vi "CRYO_MASTER_FULL_RUN3.vi"() -> ()   [LabVIEW 2017] (continued)
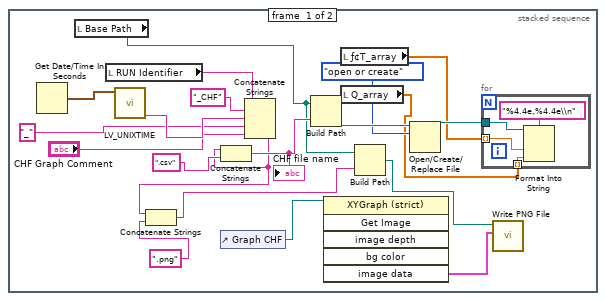
[diagram p3: hidden frame]
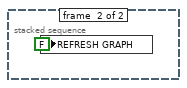
[diagram p5: hidden frame]
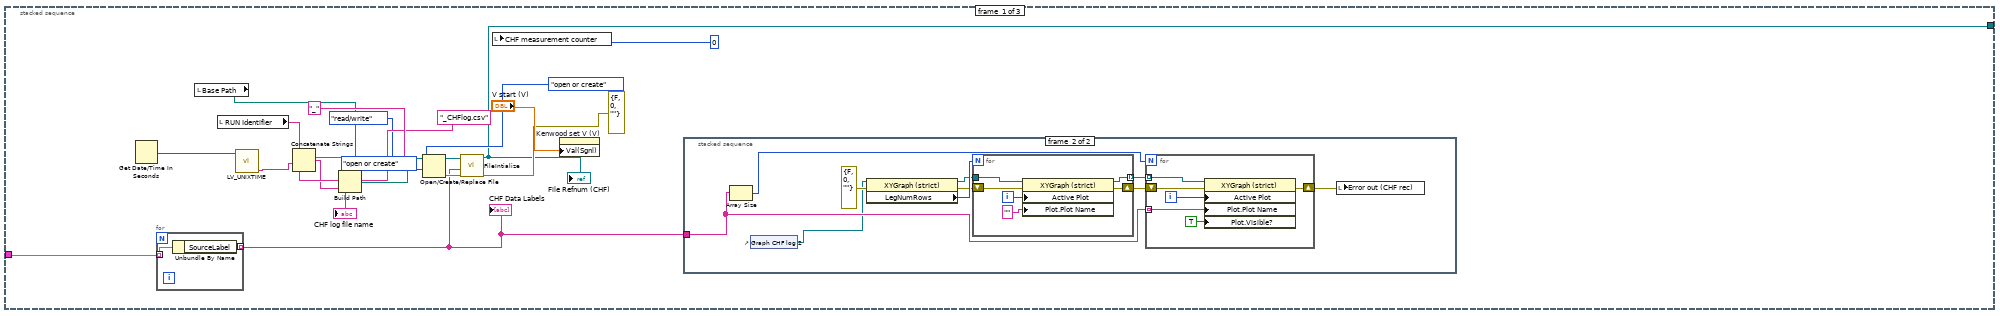
[diagram p7: hidden frame]
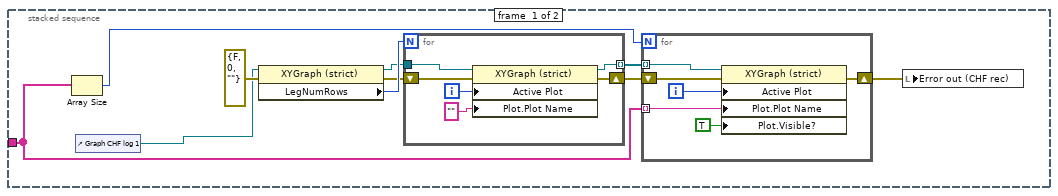
[diagram p8: hidden frame]
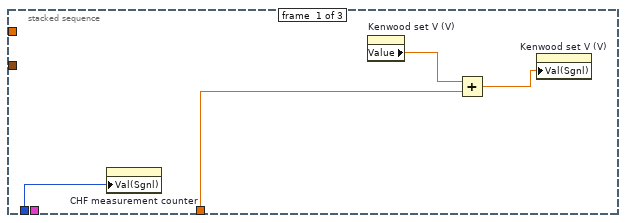
[diagram p9: hidden frame]
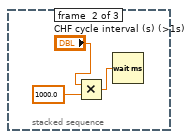
[diagram p10: hidden frame]
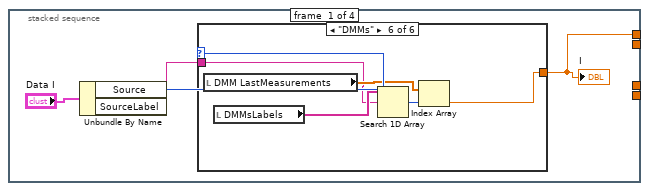
[diagram p11: hidden frame]
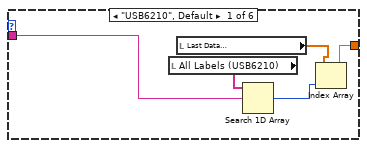
[diagram p12: hidden frame]
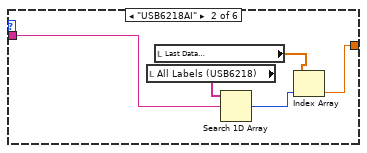
[diagram p13: hidden frame]
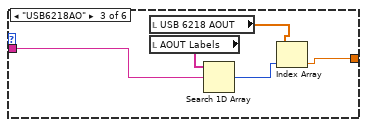
[diagram p14: hidden frame]
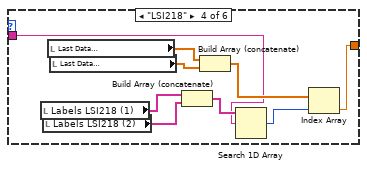
[diagram p15: hidden frame]
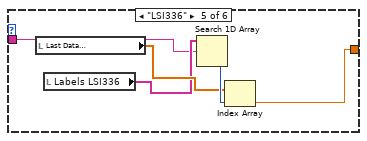
[diagram p16: hidden frame]
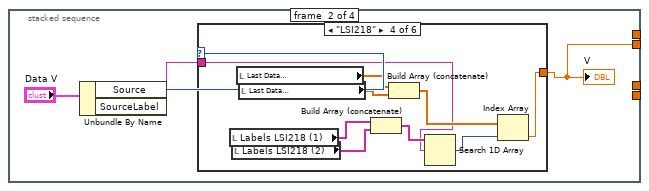
[diagram p17: hidden frame]
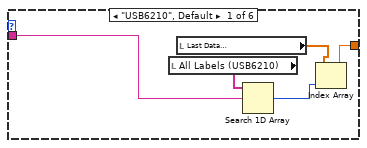
[diagram p18: hidden frame]
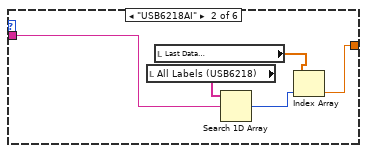
[diagram p19: hidden frame]
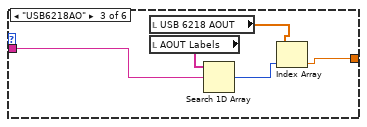
[diagram p20: hidden frame]
            frame False {
            }
            frame True {
              n984 = Build Array (concatenate)(w2040, w2041) -> (w2042:T4)
            }
          }
        }
      }
    }
    n985 = local read "Labels LSI336"() -> (w907:string[])
    n986 = Array Size(array=w907) -> (size(s)=w906:i32)
    n987 = local read "Plot selecter LSI336 \n     1      2     3     4"() -> (w915:bool[][])
    n988 = for {
      N: w906 -> [_]
      tunnel: w915 -> [w1900]
      shift-right: [w1894] -> w913
      shift-left: w914 -> [w1909]
      shift-right: [w1890] -> w912
      shift-left: w914 -> [w1907]
      shift-right: [w1891] -> w911
      shift-left: w914 -> [w1906]
      shift-right: [w1889] -> w910
      shift-left: w914 -> [w1905]
      tunnel: w876 -> [w1897]
      tunnel: w878 -> [w1895]
      i -> [w1898]
      n989 = Index Array(array=w1897, index (col)=w1898) -> (element=w1896:dbl[])  [unwired: 1 in]
      n990 = Index Array(array=w1900, index (row) #1=w1898, index (col) #1=0 ("index (row)"), index (row) #2=w1898, index (col) #2=1 ("index (row)"), index (row) #3=w1898, index (col) #3=2 ("index (row)"), index (row) #4=w1898, index (col) #4=3 ("index (row)")) -> (element #1=w1899:bool, element #2=w1893:bool, element #3=w1892:bool, element #4=w1888:bool)
      n991 = Bundle("TimeArray"=w1895, "DataArray"=w1896) -> (w1908:T35)  [unwired: 1 in]
      n992 = stacked-sequence {
        tunnel: w1909 -> [w1913 _ _ _]
        tunnel: [w1912 _ _ _] -> w1894
        tunnel: w1908 -> [w1911 w1921 w1929 w1937]
        tunnel: w1907 -> [_ w1920 _ _]
        tunnel: [_ w1919 _ _] -> w1890
        tunnel: [_ _ w1928 _] -> w1891
        tunnel: w1906 -> [_ _ w1927 _]
        tunnel: [_ _ _ w1936] -> w1889
        tunnel: w1905 -> [_ _ _ w1935]
        tunnel: w1899 -> [w1910 _ _ _]
        tunnel: w1893 -> [_ w1918 _ _]
        tunnel: w1892 -> [_ _ w1926 _]
        tunnel: w1888 -> [_ _ _ w1934]
        frame #0 {
          n993 = case shown="False" w1910 {
            tunnel: w1911 -> [_ w1915]
            tunnel: w1913 -> [w1914 w1917]
            tunnel: [w1914 w1916] -> w1912
            frame False {
            }
            frame True {
              n994 = Build Array (concatenate)(w1917, w1915) -> (w1916:T4)
            }
          }
        }
        frame #1 {
          n995 = case shown="True" w1918 {
            tunnel: [w1922 w1925] -> w1919
            tunnel: w1921 -> [_ w1923]
            tunnel: w1920 -> [w1922 w1924]
            frame False {
            }
            frame True {
              n996 = Build Array (concatenate)(w1924, w1923) -> (w1925:T4)
            }
          }
        }
        frame #2 {
          n997 = case shown="True" w1926 {
            tunnel: [w1930 w1933] -> w1928
            tunnel: w1929 -> [_ w1931]
            tunnel: w1927 -> [w1930 w1932]
            frame False {
            }
            frame True {
              n998 = Build Array (concatenate)(w1932, w1931) -> (w1933:T4)
            }
          }
        }
        frame #3 {
          n999 = case shown="True" w1934 {
            tunnel: [w1938 w1941] -> w1936
            tunnel: w1937 -> [_ w1939]
            tunnel: w1935 -> [w1938 w1940]
            frame False {
            }
            frame True {
              n1000 = Build Array (concatenate)(w1940, w1939) -> (w1941:T4)
            }
          }
        }
      }
    }
    n1001 = Array Size(array=w878) -> (size(s)=→"TimeArray Size (336)":i32)
    n1002 = Array Size(array=w876) -> (size(s)=→"DataArray size (336)":i32[])
    n1003 = Build Array (concatenate)(w932, w933, w913, w891, w836) -> (→"Graph 1":T25)
    n1004 = Build Array (concatenate)(w930, w928, w912, w890, w835) -> (→"Graph 2":T25)
    n1005 = Build Array (concatenate)(w927, w926, w911, w889, w834) -> (→"Graph 3":T25)
    n1006 = Build Array (concatenate)(w925, w924, w910, w888, w833) -> (→"Graph 4":T25)
    n1007 = Send Notification(notification="Stop Button", notifier=w853, error in (no error)=w852) -> (notifier out=w849:refnum<notifier>, error out=w850:errorcluster)
    "Cycle #" <- w842
  }
  n1008 = while {
    tunnel: w5 -> [w2130]
    tunnel: w4 -> [w2129]
    stop <- w2131 stop-if-true
    n1009 = Wait (ms)(milliseconds to wait=u32 214) -> ()  [unwired: 1 out]
    n1010 = case shown="True" "RECORD GRAPH" {
      frame False {
      }
      frame True {
        n1011 = stacked-sequence {
          frame #0 {
            n1012 = Get Date/Time In Seconds() -> (seconds since 1Jan1904=w2152:timestamp)
            n1013 = local read "Base Path"() -> (w2137:path)
            n1014 = local read "RUN Identifier"() -> (w2153:string)
            n1015 = call "LV_UNIXTIME.vi"("current time"=w2152) -> ("date/time string"=w2154:string)  [unwired: 9 in, 1 out]
            n1016 = control-ref of="Graph CHF"() -> (w2143:refnum<vi>)
            n1017 = Concatenate Strings(w2153, "_CHF" ("string"), w2154, "_" ("string"), "CHF Graph Comment") -> (w2139:string)
            n1018 = Concatenate Strings(w2139, ".png" ("string")) -> (w2138:string)
            n1019 = Concatenate Strings(w2139, ".csv" ("string")) -> (w2141:string)
            "CHF file name" <- w2141
            n1020 = Build Path(base path=w2137, name or relative path=w2141) -> (appended path=w2148:path)
            n1021 = invoke class="XYGraph (strict)" method="Get Image"(reference=w2143) -> ("image data"=w2135:T23)  [unwired: 5 in, 5 out]
            n1022 = local read "ƒ¢T_array"() -> (w2145:dbl[])
            n1023 = local read "Q_array"() -> (w2144:dbl[])
            n1024 = Build Path(base path=w2137, name or relative path=w2138) -> (appended path=w2136:path)
            n1025 = Open/Create/Replace File(file path (use dialog)=w2148, operation (0:open)=T24."open or create") -> (refnum out=w2146:refnum<file>)  [unwired: 4 in, 2 out]
            n1026 = for {
              tunnel: w2146 -> [w2158]
              tunnel: w2145 -> [w2156] mode=indexing
              tunnel: w2144 -> [w2155] mode=indexing
              n1027 = Format Into String(format string="%4.4e,%4.4e\\n" ("prompt"), initial string=w2158, w2156, w2155) -> ()  [unwired: 1 in, 2 out]
            }
            n1028 = call <vilib>:"Write PNG File.vi"("image data"=w2135, "path to PNG file"=w2136) -> ()  [unwired: 8 in, 2 out]
          }
          frame #1 {
            n1029 = local write "RECORD GRAPH"(FALSE ("RECORD GRAPH")) -> ()
          }
        }
      }
    }
    n1030 = case shown="True" "START CHF" {
      tunnel: "RecordSettings" -> [_ w2163]
      frame False {
      }
      frame True {
        n1031 = stacked-sequence {
          tunnel: [w2167 _ _] -> _
          tunnel: w2163 -> [w2166 w2240 _]
          frame #0 {
            (unwired) T24."open or create" ("operation (0:open)")
            n1032 = Get Date/Time In Seconds() -> (seconds since 1Jan1904=w2179:timestamp)
            n1033 = for {
              tunnel: [w2227] -> w2165 mode=indexing
              tunnel: w2166 -> [w2226] mode=indexing
              n1034 = Unbundle By Name(w2226) -> ("SourceLabel"=w2227:string)
            }
            "CHF Data Labels" <- w2165
            n1035 = local read "Base Path"() -> (w2174:path)
            n1036 = local read "RUN Identifier"() -> (w2178:string)
            n1037 = call "LV_UNIXTIME.vi"("current time"=w2179) -> ("date/time string"=w2177:string)  [unwired: 9 in, 1 out]
            n1038 = Concatenate Strings(w2178, "_" ("string"), w2177, "_CHFlog.csv" ("string")) -> (w2173:string)
            "CHF log file name" <- w2173
            n1039 = Build Path(base path=w2174, name or relative path=w2173) -> (appended path=w2172:path)
            n1040 = Open/Create/Replace File(file path (use dialog)=w2172, error in=errorcluster {"status"=FALSE, "code"=0, "source"=""}, operation (0:open)=T24."open or create", access (0:read/write)=enum16{"read/write", "read-only", "write-only"}."read/write") -> (refnum out=w2170:refnum<file>, error out=w2169:errorcluster)  [unwired: 2 in, 1 out]
            n1041 = call "FileIntialize.vi"("Error In"=w2169, "Labels"=w2165, "refnum in"=w2170) -> ("File Refnum"=w2167:refnum<file>)  [unwired: 7 in, 1 out]
            "File Refnum (CHF)" <- w2167
            n1042 = local write "CHF measurement counter"(0 ("CHF counter")) -> ()
            n1043 = property on="Kenwood set V (V)" class="DigNum (strict)"("Val(Sgnl)"="V start (V)") -> ()  [unwired: 2 in, 2 out]
            n1044 = stacked-sequence {
              tunnel: w2165 -> [w2183 w2206]
              frame #0 {
                n1045 = Array Size(array=w2183) -> (size(s)=w2191:i32)
                n1046 = control-ref of="Graph CHF log 1"() -> (w2184:refnum<vi>)
                n1047 = property class="XYGraph (strict)"(reference=w2184, error in=errorcluster {"status"=FALSE, "code"=0, "source"=""} ("error in (no error)")) -> (reference out=w2186:refnum<vi>, error out=w2188:errorcluster, "LegNumRows"=w2189:u32)
                n1048 = for {
                  N: w2189 -> [_]
                  shift-right: [w2200] -> w2190
                  shift-left: w2188 -> [w2201]
                  tunnel: w2186 -> [w2199]
                  tunnel: [w2198] -> w2185 mode=indexing
                  i -> [w2203]
                  n1049 = property class="XYGraph (strict)"(reference=w2199, error in=w2201, "Active Plot"=w2203, "Plot.Plot Name"="") -> (reference out=w2198:refnum<vi>, error out=w2200:errorcluster)
                }
                n1050 = for {
                  N: w2191 -> [_]
                  shift-right: [w2195] -> w2182
                  shift-left: w2190 -> [w2196]
                  tunnel: w2185 -> [w2193] mode=indexing
                  tunnel: w2183 -> [w2192] mode=indexing
                  i -> [w2197]
                  n1051 = property class="XYGraph (strict)"(reference=w2193, error in=w2196, "Active Plot"=w2197, "Plot.Plot Name"=w2192, "Plot.Visible?"=TRUE ("Plot.Visible")) -> (error out=w2195:errorcluster)  [unwired: 1 out]
                }
                n1052 = local write "Error out (CHF rec)"(w2182) -> ()
              }
              frame #1 {
                n1053 = Array Size(array=w2206) -> (size(s)=w2213:i32)
                n1054 = control-ref of="Graph CHF log 2"() -> (w2205:refnum<vi>)
                n1055 = property class="XYGraph (strict)"(reference=w2205, error in=errorcluster {"status"=FALSE, "code"=0, "source"=""} ("error in (no error)")) -> (reference out=w2208:refnum<vi>, error out=w2210:errorcluster, "LegNumRows"=w2211:u32)
                n1056 = for {
                  N: w2211 -> [_]
                  shift-right: [w2222] -> w2212
                  shift-left: w2210 -> [w2223]
                  tunnel: w2208 -> [w2221]
                  tunnel: [w2220] -> w2207 mode=indexing
                  i -> [w2225]
                  n1057 = property class="XYGraph (strict)"(reference=w2221, error in=w2223, "Active Plot"=w2225, "Plot.Plot Name"="") -> (reference out=w2220:refnum<vi>, error out=w2222:errorcluster)
                }
                n1058 = for {
                  N: w2213 -> [_]
                  shift-right: [w2217] -> w2204
                  shift-left: w2212 -> [w2218]
                  tunnel: w2207 -> [w2215] mode=indexing
                  tunnel: w2206 -> [w2214] mode=indexing
                  i -> [w2219]
                  n1059 = property class="XYGraph (strict)"(reference=w2215, error in=w2218, "Active Plot"=w2219, "Plot.Plot Name"=w2214, "Plot.Visible?"=TRUE ("Plot.Visible")) -> (error out=w2217:errorcluster)  [unwired: 1 out]
                }
                n1060 = local write "Error out (CHF rec)"(w2204) -> ()
              }
            }
          }
          frame #1 {
            n1061 = local read "V start (V)"() -> (w2239:dbl)
            n1062 = Absolute Value(x="V_end (V)") -> (abs(x)=w2236:dbl)
            n1063 = Absolute Value(x=w2239) -> (abs(x)=w2237:dbl)
            n1064 = Build Array(w2237, w2236) -> (w2235:dbl[])
            n1065 = Array Max & Min(array=w2235) -> (max value=w2234:dbl, min value=w2233:dbl)  [unwired: 2 out]
            n1066 = Subtract(x=w2234, y=w2233) -> (x-y=w2232:dbl)
            n1067 = Quotient & Remainder(x=w2232, y="ƒ¢V / cycle (V)") -> (floor(x/y)=w2230:dbl)  [unwired: 1 out]
            n1068 = for {
              N: w2230 -> [_]
              tunnel: w2240 -> [w2248]
              shift-right: [w2244] -> _
              shift-left: dbl[][] [] -> [w2246]
              shift-right: [w2243] -> _
              shift-left: timestamp[] [] -> [w2245]
              tunnel: "ƒ¢V / cycle (V)" -> [w2242]
              i -> [w2247]
              n1069 = case shown="False" "STOP CHF" {
                tunnel: w2248 -> [w2264 _]
                tunnel: w2247 -> [w2263 _]
                tunnel: w2246 -> [w2262 w2489]
                tunnel: w2245 -> [w2258 w2488]
                tunnel: [w2255 w2489] -> w2244
                tunnel: [w2254 w2488] -> w2243
                tunnel: w2242 -> [w2249 _]
                frame False {
                  n1070 = stacked-sequence {
                    tunnel: w2264 -> [_ _ w2296]
                    tunnel: [_ _ w2287] -> w2253
                    tunnel: w2263 -> [_ _ w2286]
                    tunnel: w2263 -> [w2271 _ _]
                    tunnel: [_ _ w2284] -> w2252
                    tunnel: [_ _ w2283] -> w2257
                    tunnel: [_ _ w2282] -> w2261
                    tunnel: w2262 -> [_ _ w2282]
                    tunnel: [_ _ w2281] -> w2260
                    tunnel: w2258 -> [_ _ w2280]
                    tunnel: [_ _ w2280] -> w2259
                    tunnel: w2249 -> [w2270 _ _]
                    frame #0 {
                      n1071 = property on="CHF measurement counter" class="DigNum (strict)"("Val(Sgnl)"=w2271) -> ()  [unwired: 2 in, 2 out]
                      n1072 = property on="Kenwood set V (V)" class="DigNum (strict)"() -> ("Value"=w2273:dbl)  [unwired: 2 in, 2 out]
                      n1073 = Add(x=w2273, y=w2270) -> (x+y=w2272:dbl)
                      n1074 = property on="Kenwood set V (V)" class="DigNum (strict)"("Val(Sgnl)"=w2272) -> ()  [unwired: 2 in, 2 out]
                    }
                    frame #1 {
                      n1075 = Multiply(x="CHF cycle interval (s) (>1s)", y=1000.0) -> (x*y=w2275:dbl)
                      n1076 = Wait (ms)(milliseconds to wait=w2275) -> ()  [unwired: 1 out]
                    }
                    frame #2 {
                      n1077 = for {
                        tunnel: w2296 -> [w2453] mode=indexing
                        tunnel: [w2451] -> w2283 mode=indexing
                        tunnel: [w2449] -> w2294 mode=indexing
                        n1078 = Unbundle By Name(w2453) -> ("Source"=w2452:T36, "SourceLabel"=w2450:string, "FileFormat"=w2449:string)
                        n1079 = case shown="\"LSI218\"" w2452 {
                          tunnel: [w2454 w2459 w2464 w2470 w2478 w2483] -> w2451
                          tunnel: w2450 -> [w2455 w2461 w2466 w2469 w2479 w2487]
                          frame "USB6210", Default {
                            n1080 = local read "All Labels (USB6210)"() -> (w2457:string[])
                            n1081 = local read "Last Data \n(USB6210)"() -> (w2458:dbl[])
                            n1082 = Search 1D Array(1D array=w2457, element=w2455) -> (index of element=w2456:i32)  [unwired: 1 in]
                            n1083 = Index Array(array=w2458, index=w2456) -> (element=w2454:dbl)
                          }
                          frame "USB6218AI" {
                            n1084 = local read "All Labels (USB6218)"() -> (w2462:string[])
                            n1085 = local read "Last Data \n(USB6218)"() -> (w2463:dbl[])
                            n1086 = Search 1D Array(1D array=w2462, element=w2461) -> (index of element=w2460:i32)  [unwired: 1 in]
                            n1087 = Index Array(array=w2463, index=w2460) -> (element=w2459:dbl)
                          }
                          frame "USB6218AO" {
                            n1088 = local read "USB 6218 AOUT"() -> (w2468:dbl[])
                            n1089 = local read "AOUT Labels"() -> (w2467:string[])
                            n1090 = Search 1D Array(1D array=w2467, element=w2466) -> (index of element=w2465:i32)  [unwired: 1 in]
                            n1091 = Index Array(array=w2468, index=w2465) -> (element=w2464:dbl)
                          }
                          frame "LSI218" {
                            n1092 = local read "Labels LSI218 (1)"() -> (w2473:string[])
                            n1093 = local read "Labels LSI218 (2)"() -> (w2472:string[])
                            n1094 = local read "Last Data \nLSI218 (1)"() -> (w2476:dbl[])
                            n1095 = local read "Last Data \nLSI218 (2)"() -> (w2475:dbl[])
                            n1096 = Build Array (concatenate)(w2473, w2472) -> (w2471:string[])
                            n1097 = Build Array (concatenate)(w2476, w2475) -> (w2474:dbl[])
                            n1098 = Search 1D Array(1D array=w2471, element=w2469) -> (index of element=w2477:i32)  [unwired: 1 in]
                            n1099 = Index Array(array=w2474, index=w2477) -> (element=w2470:dbl)
                          }
                          frame "LSI336" {
                            n1100 = local read "Last Data \nLSI336"() -> (w2481:dbl[])
                            n1101 = local read "Labels LSI336"() -> (w2482:string[])
                            n1102 = Search 1D Array(1D array=w2482, element=w2479) -> (index of element=w2480:i32)  [unwired: 1 in]
                            n1103 = Index Array(array=w2481, index=w2480) -> (element=w2478:dbl)
                          }
                          frame "DMMs" {
                            n1104 = local read "DMM LastMeasurements"() -> (w2484:dbl[])
                            n1105 = local read "DMMsLabels"() -> (w2486:string[])
                            n1106 = Search 1D Array(1D array=w2486, element=w2487) -> (index of element=w2485:i32)  [unwired: 1 in]
                            n1107 = Index Array(array=w2484, index=w2485) -> (element=w2483:dbl)
                          }
                        }
                      }
                      "CHF last data" <- w2283
                      n1108 = stacked-sequence {
                        tunnel: [w2297 _ _ _] -> w2292
                        tunnel: [_ w2335 _ _] -> w2291
                        tunnel: [_ _ _ w2411] -> w2290
                        tunnel: [_ _ w2373 _] -> w2289
                        frame #0 {
                          n1109 = Unbundle By Name("Data I") -> ("Source"=w2299:T36, "SourceLabel"=w2298:string)
                          n1110 = case shown="\"DMMs\"" w2299 {
                            tunnel: w2298 -> [w2302 w2307 w2312 w2317 w2326 w2331]
                            tunnel: [w2301 w2306 w2311 w2316 w2325 w2330] -> w2297
                            frame "USB6210", Default {
                              n1111 = local read "All Labels (USB6210)"() -> (w2304:string[])
                              n1112 = local read "Last Data \n(USB6210)"() -> (w2303:dbl[])
                              n1113 = Search 1D Array(1D array=w2304, element=w2302) -> (index of element=w2305:i32)  [unwired: 1 in]
                              n1114 = Index Array(array=w2303, index=w2305) -> (element=w2301:dbl)
                            }
                            frame "USB6218AI" {
                              n1115 = local read "All Labels (USB6218)"() -> (w2309:string[])
                              n1116 = local read "Last Data \n(USB6218)"() -> (w2308:dbl[])
                              n1117 = Search 1D Array(1D array=w2309, element=w2307) -> (index of element=w2310:i32)  [unwired: 1 in]
                              n1118 = Index Array(array=w2308, index=w2310) -> (element=w2306:dbl)
                            }
                            frame "USB6218AO" {
                              n1119 = local read "USB 6218 AOUT"() -> (w2313:dbl[])
                              n1120 = local read "AOUT Labels"() -> (w2314:string[])
                              n1121 = Search 1D Array(1D array=w2314, element=w2312) -> (index of element=w2315:i32)  [unwired: 1 in]
                              n1122 = Index Array(array=w2313, index=w2315) -> (element=w2311:dbl)
                            }
                            frame "LSI218" {
                              n1123 = local read "Labels LSI218 (1)"() -> (w2322:string[])
                              n1124 = local read "Labels LSI218 (2)"() -> (w2323:string[])
                              n1125 = local read "Last Data \nLSI218 (1)"() -> (w2319:dbl[])
                              n1126 = local read "Last Data \nLSI218 (2)"() -> (w2320:dbl[])
                              n1127 = Build Array (concatenate)(w2322, w2323) -> (w2324:string[])
                              n1128 = Build Array (concatenate)(w2319, w2320) -> (w2321:dbl[])
                              n1129 = Search 1D Array(1D array=w2324, element=w2317) -> (index of element=w2318:i32)  [unwired: 1 in]
                              n1130 = Index Array(array=w2321, index=w2318) -> (element=w2316:dbl)
                            }
                            frame "LSI336" {
                              n1131 = local read "Last Data \nLSI336"() -> (w2328:dbl[])
                              n1132 = local read "Labels LSI336"() -> (w2327:string[])
                              n1133 = Search 1D Array(1D array=w2327, element=w2326) -> (index of element=w2329:i32)  [unwired: 1 in]
                              n1134 = Index Array(array=w2328, index=w2329) -> (element=w2325:dbl)
                            }
                            frame "DMMs" {
                              n1135 = local read "DMM LastMeasurements"() -> (w2334:dbl[])
                              n1136 = local read "DMMsLabels"() -> (w2332:string[])
                              n1137 = Search 1D Array(1D array=w2332, element=w2331) -> (index of element=w2333:i32)  [unwired: 1 in]
                              n1138 = Index Array(array=w2334, index=w2333) -> (element=w2330:dbl)
                            }
                          }
                          "I" <- w2297
                        }
                        frame #1 {
                          n1139 = Unbundle By Name("Data V") -> ("Source"=w2338:T36, "SourceLabel"=w2337:string)
                          n1140 = case shown="\"LSI218\"" w2338 {
                            tunnel: w2337 -> [w2340 w2345 w2350 w2355 w2364 w2369]
                            tunnel: [w2339 w2344 w2349 w2354 w2363 w2368] -> w2335
                            frame "USB6210", Default {
                              n1141 = local read "All Labels (USB6210)"() -> (w2342:string[])
                              n1142 = local read "Last Data \n(USB6210)"() -> (w2341:dbl[])
                              n1143 = Search 1D Array(1D array=w2342, element=w2340) -> (index of element=w2343:i32)  [unwired: 1 in]
                              n1144 = Index Array(array=w2341, index=w2343) -> (element=w2339:dbl)
                            }
                            frame "USB6218AI" {
                              n1145 = local read "All Labels (USB6218)"() -> (w2347:string[])
                              n1146 = local read "Last Data \n(USB6218)"() -> (w2346:dbl[])
                              n1147 = Search 1D Array(1D array=w2347, element=w2345) -> (index of element=w2348:i32)  [unwired: 1 in]
                              n1148 = Index Array(array=w2346, index=w2348) -> (element=w2344:dbl)
                            }
                            frame "USB6218AO" {
                              n1149 = local read "USB 6218 AOUT"() -> (w2351:dbl[])
                              n1150 = local read "AOUT Labels"() -> (w2352:string[])
                              n1151 = Search 1D Array(1D array=w2352, element=w2350) -> (index of element=w2353:i32)  [unwired: 1 in]
                              n1152 = Index Array(array=w2351, index=w2353) -> (element=w2349:dbl)
                            }
                            frame "LSI218" {
                              n1153 = local read "Labels LSI218 (1)"() -> (w2360:string[])
                              n1154 = local read "Labels LSI218 (2)"() -> (w2361:string[])
                              n1155 = local read "Last Data \nLSI218 (1)"() -> (w2357:dbl[])
                              n1156 = local read "Last Data \nLSI218 (2)"() -> (w2358:dbl[])
                              n1157 = Build Array (concatenate)(w2360, w2361) -> (w2362:string[])
                              n1158 = Build Array (concatenate)(w2357, w2358) -> (w2359:dbl[])
                              n1159 = Search 1D Array(1D array=w2362, element=w2355) -> (index of element=w2356:i32)  [unwired: 1 in]
                              n1160 = Index Array(array=w2359, index=w2356) -> (element=w2354:dbl)
                            }
                            frame "LSI336" {
                              n1161 = local read "Last Data \nLSI336"() -> (w2366:dbl[])
                              n1162 = local read "Labels LSI336"() -> (w2365:string[])
                              n1163 = Search 1D Array(1D array=w2365, element=w2364) -> (index of element=w2367:i32)  [unwired: 1 in]
                              n1164 = Index Array(array=w2366, index=w2367) -> (element=w2363:dbl)
                            }
                            frame "DMMs" {
                              n1165 = local read "DMM LastMeasurements"() -> (w2372:dbl[])
                              n1166 = local read "DMMsLabels"() -> (w2370:string[])
                              n1167 = Search 1D Array(1D array=w2370, element=w2369) -> (index of element=w2371:i32)  [unwired: 1 in]
                              n1168 = Index Array(array=w2372, index=w2371) -> (element=w2368:dbl)
                            }
                          }
                          "V" <- w2335
                        }
                        frame #2 {
                          n1169 = Unbundle By Name("Data T_low") -> ("Source"=w2376:T36, "SourceLabel"=w2375:string)
                          n1170 = case shown="\"DMMs\"" w2376 {
                            tunnel: w2375 -> [w2378 w2383 w2388 w2393 w2402 w2407]
                            tunnel: [w2377 w2382 w2387 w2392 w2401 w2406] -> w2373
                            frame "USB6210", Default {
                              n1171 = local read "All Labels (USB6210)"() -> (w2380:string[])
                              n1172 = local read "Last Data \n(USB6210)"() -> (w2379:dbl[])
                              n1173 = Search 1D Array(1D array=w2380, element=w2378) -> (index of element=w2381:i32)  [unwired: 1 in]
                              n1174 = Index Array(array=w2379, index=w2381) -> (element=w2377:dbl)
                            }
                            frame "USB6218AI" {
                              n1175 = local read "All Labels (USB6218)"() -> (w2385:string[])
                              n1176 = local read "Last Data \n(USB6218)"() -> (w2384:dbl[])
                              n1177 = Search 1D Array(1D array=w2385, element=w2383) -> (index of element=w2386:i32)  [unwired: 1 in]
                              n1178 = Index Array(array=w2384, index=w2386) -> (element=w2382:dbl)
                            }
                            frame "USB6218AO" {
                              n1179 = local read "USB 6218 AOUT"() -> (w2389:dbl[])
                              n1180 = local read "AOUT Labels"() -> (w2390:string[])
                              n1181 = Search 1D Array(1D array=w2390, element=w2388) -> (index of element=w2391:i32)  [unwired: 1 in]
                              n1182 = Index Array(array=w2389, index=w2391) -> (element=w2387:dbl)
                            }
                            frame "LSI218" {
                              n1183 = local read "Labels LSI218 (1)"() -> (w2398:string[])
                              n1184 = local read "Labels LSI218 (2)"() -> (w2399:string[])
                              n1185 = local read "Last Data \nLSI218 (1)"() -> (w2395:dbl[])
                              n1186 = local read "Last Data \nLSI218 (2)"() -> (w2396:dbl[])
                              n1187 = Build Array (concatenate)(w2398, w2399) -> (w2400:string[])
                              n1188 = Build Array (concatenate)(w2395, w2396) -> (w2397:dbl[])
                              n1189 = Search 1D Array(1D array=w2400, element=w2393) -> (index of element=w2394:i32)  [unwired: 1 in]
                              n1190 = Index Array(array=w2397, index=w2394) -> (element=w2392:dbl)
                            }
                            frame "LSI336" {
                              n1191 = local read "Last Data \nLSI336"() -> (w2404:dbl[])
                              n1192 = local read "Labels LSI336"() -> (w2403:string[])
                              n1193 = Search 1D Array(1D array=w2403, element=w2402) -> (index of element=w2405:i32)  [unwired: 1 in]
                              n1194 = Index Array(array=w2404, index=w2405) -> (element=w2401:dbl)
                            }
                            frame "DMMs" {
                              n1195 = local read "DMM LastMeasurements"() -> (w2410:dbl[])
                              n1196 = local read "DMMsLabels"() -> (w2408:string[])
                              n1197 = Search 1D Array(1D array=w2408, element=w2407) -> (index of element=w2409:i32)  [unwired: 1 in]
                              n1198 = Index Array(array=w2410, index=w2409) -> (element=w2406:dbl)
                            }
                          }
                          "T_low" <- w2373
                        }
                        frame #3 {
                          n1199 = Unbundle By Name("Data T_high") -> ("Source"=w2414:T36, "SourceLabel"=w2413:string)
                          n1200 = case shown="\"DMMs\"" w2414 {
                            tunnel: w2413 -> [w2416 w2421 w2426 w2431 w2440 w2445]
                            tunnel: [w2415 w2420 w2425 w2430 w2439 w2444] -> w2411
                            frame "USB6210", Default {
                              n1201 = local read "All Labels (USB6210)"() -> (w2418:string[])
                              n1202 = local read "Last Data \n(USB6210)"() -> (w2417:dbl[])
                              n1203 = Search 1D Array(1D array=w2418, element=w2416) -> (index of element=w2419:i32)  [unwired: 1 in]
                              n1204 = Index Array(array=w2417, index=w2419) -> (element=w2415:dbl)
                            }
                            frame "USB6218AI" {
                              n1205 = local read "All Labels (USB6218)"() -> (w2423:string[])
                              n1206 = local read "Last Data \n(USB6218)"() -> (w2422:dbl[])
                              n1207 = Search 1D Array(1D array=w2423, element=w2421) -> (index of element=w2424:i32)  [unwired: 1 in]
                              n1208 = Index Array(array=w2422, index=w2424) -> (element=w2420:dbl)
                            }
                            frame "USB6218AO" {
                              n1209 = local read "USB 6218 AOUT"() -> (w2427:dbl[])
                              n1210 = local read "AOUT Labels"() -> (w2428:string[])
                              n1211 = Search 1D Array(1D array=w2428, element=w2426) -> (index of element=w2429:i32)  [unwired: 1 in]
                              n1212 = Index Array(array=w2427, index=w2429) -> (element=w2425:dbl)
                            }
                            frame "LSI218" {
                              n1213 = local read "Labels LSI218 (1)"() -> (w2436:string[])
                              n1214 = local read "Labels LSI218 (2)"() -> (w2437:string[])
                              n1215 = local read "Last Data \nLSI218 (1)"() -> (w2433:dbl[])
                              n1216 = local read "Last Data \nLSI218 (2)"() -> (w2434:dbl[])
                              n1217 = Build Array (concatenate)(w2436, w2437) -> (w2438:string[])
                              n1218 = Build Array (concatenate)(w2433, w2434) -> (w2435:dbl[])
                              n1219 = Search 1D Array(1D array=w2438, element=w2431) -> (index of element=w2432:i32)  [unwired: 1 in]
                              n1220 = Index Array(array=w2435, index=w2432) -> (element=w2430:dbl)
                            }
                            frame "LSI336" {
                              n1221 = local read "Last Data \nLSI336"() -> (w2442:dbl[])
                              n1222 = local read "Labels LSI336"() -> (w2441:string[])
                              n1223 = Search 1D Array(1D array=w2441, element=w2440) -> (index of element=w2443:i32)  [unwired: 1 in]
                              n1224 = Index Array(array=w2442, index=w2443) -> (element=w2439:dbl)
                            }
                            frame "DMMs" {
                              n1225 = local read "DMM LastMeasurements"() -> (w2448:dbl[])
                              n1226 = local read "DMMsLabels"() -> (w2446:string[])
                              n1227 = Search 1D Array(1D array=w2446, element=w2445) -> (index of element=w2447:i32)  [unwired: 1 in]
                              n1228 = Index Array(array=w2448, index=w2447) -> (element=w2444:dbl)
                            }
                          }
                          "T_high" <- w2411
                        }
                      }
                      n1229 = local read "File Refnum (CHF)"() -> (w2277:refnum<file>)
                      n1230 = Get Date/Time In Seconds() -> (seconds since 1Jan1904=w2281:timestamp)
                      n1231 = Subtract(x=w2290, y=w2289) -> (x-y=w2285:dbl)
                      "ƒ¢T" <- w2285
                      n1232 = Multiply(x=w2292, y=w2291) -> (x*y=w2288:dbl)
                      "Q" <- w2288
                      n1233 = local read "ƒ¢T_array"() -> (w2279:dbl[])
                      n1234 = local read "Q_array"() -> (w2278:dbl[])
                      n1235 = call "FileWrite.vi"("DataArray"=w2283, "Time Stamp"=w2281, "Error In"=errorcluster {"status"=FALSE, "code"=0, "source"=""}, "FileFormat"=w2294, "Index"=w2286, "refnum in"=w2277) -> ("Error Out"=→"Error out (CHF rec)":errorcluster)  [unwired: 4 in, 1 out]
                      n1236 = Build Array (concatenate)(w2279, w2285) -> (w2284:dbl[])
                      n1237 = Build Array (concatenate)(w2278, w2288) -> (w2287:dbl[])
                    }
                  }
                  n1238 = Build Array (concatenate)(w2261, w2257) -> (w2255:dbl[][])
                  n1239 = Build Array (concatenate)(w2259, w2260) -> (w2254:timestamp[])
                  n1240 = Bundle(w2252, w2253) -> (→"Graph CHF":cluster{dbl[], dbl[]})  [unwired: 1 in]
                  n1241 = local write "ƒ¢T_array"(w2252) -> ()
                  n1242 = local write "Q_array"(w2253) -> ()
                  n1243 = Array Size(array=w2257) -> (size(s)=w2256:i32)
                  n1244 = for {
                    N: w2256 -> [_]
                    tunnel: w2255 -> [w2269]
                    tunnel: w2254 -> [w2267]
                    tunnel: [w2265] -> w2250 mode=indexing
                    i -> [w2268]
                    n1245 = Index Array(array=w2269, index (col)=w2268) -> (element=w2266:dbl[])  [unwired: 1 in]
                    n1246 = Bundle(w2267, w2266) -> (w2265:cluster{timestamp[], dbl[]})  [unwired: 1 in]
                  }
                  "Graph CHF log 2" <- w2250
                  "Graph CHF log 1" <- w2250
                  "Graph CHF log 3" <- w2250
                }
                frame True {
                }
              }
            }
          }
          frame #2 {
            n1247 = local write "CHF measurement counter"(0 ("CHF counter")) -> ()
            n1248 = local write "START CHF"(FALSE ("START CHF")) -> ()
            n1249 = local write "STOP CHF"(FALSE ("STOP CHF")) -> ()
          }
        }
      }
    }
    n1250 = case shown="True" "REFRESH GRAPH" {
      frame False {
      }
      frame True {
        n1251 = stacked-sequence {
          frame #0 {
            w2161 = dbl[] [] ("ƒ¢T_array")
            n1252 = local write "ƒ¢T_array"(w2161) -> ()
            n1253 = local write "Q_array"(w2161) -> ()
            n1254 = Bundle("ƒ¢T_array"=w2161, "ƒ¢T_array"=w2161) -> (w2160:cluster{"ƒ¢T_array":dbl[], "ƒ¢T_array":dbl[]})  [unwired: 1 in]
            n1255 = local write "Graph CHF"(w2160) -> ()
          }
          frame #1 {
            n1256 = local write "REFRESH GRAPH"(FALSE ("REFRESH GRAPH")) -> ()
          }
        }
      }
    }
    n1257 = Get Notifier Status(notifier=w2130, error in (no error)=w2129) -> (current notification=w2131:bool)  [unwired: 4 out]
  }
  n1258 = while {
    shift-right: [w2502] -> w8
    shift-left: refnum<class "DMMsData.lvclass"> refnum ("DMMsData.lvclass") -> [w2501]
    shift-right: [w2500] -> w7
    shift-left: errorcluster {"status"=FALSE, "code"=0, "source"=""} ("error in (no error)") -> [w2493]
    tunnel: w5 -> [w2498]
    tunnel: w4 -> [w2497]
    tunnel: [w2496] -> w11
    i -> [w2499]
    stop <- w2495 stop-if-true
    n1259 = Equal?(x=w2499, y=0) -> (x = y?=w2503:bool)
    n1260 = Wait (ms)(milliseconds to wait="Measurement Interval DMMs (ms)") -> ()  [unwired: 1 out]
    n1261 = case shown="True" "Measure DMMs?" {
      tunnel: w2503 -> [_ w2514]
      tunnel: [w2507 w2512] -> w2502
      tunnel: w2501 -> [w2507 w2511]
      tunnel: w2493 -> [w2506 w2510]
      tunnel: [w2506 w2509] -> w2500
      tunnel: w2499 -> [_ w2508]
      frame False {
      }
      frame True {
        n1262 = Or(x="Initialize (DMMs)", y=w2514) -> (x .or. y?=w2513:bool)
        n1263 = case shown="False" w2513 {
          tunnel: w2511 -> [w2545 w2581]
          tunnel: [w2542 w2580] -> w2512
          tunnel: w2510 -> [w2544 w2577]
          tunnel: [w2543 w2574] -> w2509
          tunnel: w2508 -> [w2541 _]
          frame False {
            n1264 = local read "VariableSources"() -> (w2534:T12)
            n1265 = for {
              tunnel: w2534 -> [w2548] mode=indexing
              tunnel: [w2547] -> w2533 mode=indexing
              tunnel: [w2546] -> w2532 mode=indexing
              n1266 = case shown="\"LSI218\"" w2548 {
                tunnel: [w2550 w2552 w2554 w2555 w2561] -> w2547
                tunnel: [w2549 w2551 w2553 w2556 w2562] -> w2546
                frame "USB6210" {
                  n1267 = local read "All Labels (USB6210)"() -> (w2550:string[])
                  n1268 = local read "Last Data \n(USB6210)"() -> (w2549:dbl[])
                }
                frame "USB6218AI" {
                  n1269 = local read "Last Data \n(USB6218)"() -> (w2551:dbl[])
                  n1270 = local read "All Labels (USB6218)"() -> (w2552:string[])
                }
                frame "USB6218AO" {
                  n1271 = local read "USB 6218 AOUT"() -> (w2553:dbl[])
                  n1272 = local read "AOUT Labels"() -> (w2554:string[])
                }
                frame "LSI218" {
                  n1273 = local read "Last Data \nLSI218 (2)"() -> (w2557:dbl[])
                  n1274 = local read "Last Data \nLSI218 (1)"() -> (w2558:dbl[])
                  n1275 = local read "Labels LSI218 (2)"() -> (w2560:string[])
                  n1276 = local read "Labels LSI218 (1)"() -> (w2559:string[])
                  n1277 = Build Array (concatenate)(w2558, w2557) -> (w2556:dbl[])
                  n1278 = Build Array (concatenate)(w2559, w2560) -> (w2555:string[])
                }
                frame "LSI336" {
                  n1279 = local read "Last Data \nLSI336"() -> (w2562:dbl[])
                  n1280 = local read "Labels LSI336"() -> (w2561:string[])
                }
              }
            }
            n1281 = local read "DMMsConfig (variables)"() -> (w2526:T13)
            n1282 = local read "DMMsConfig"() -> (w2538:T11)
            n1283 = call-dynamic "DMMs_measure.vi"("DMMsData in"=w2545, "Sample #"="Sample #", "MeasurementIndex"=w2541, "SourceDataLabels"=w2533, "error in (no error)"=w2544, "SourceDataArray"=w2532) -> ("TimeArray"=w2540:timestamp[], "DMMsData out"=w2542:refnum<class "DMMsData.lvclass">, "LastData"=w2520:dbl[], "DataArray"=w2537:dbl[][], "DeviceActive?"=→"Active?":bool[], "error out"=w2543:errorcluster)  [unwired: 4 in]
            "DMM LastMeasurements" <- w2520
            n1284 = Array Size(array=w2526) -> (size(s)=w2524:i32)
            n1285 = Array Size(array=w2538) -> (size(s)=w2525:i32)
            n1286 = Add(x=w2525, y=w2524) -> (x+y=w2523:i32)
            n1287 = for {
              N: w2523 -> [_]
              tunnel: w2540 -> [w2565]
              tunnel: w2537 -> [w2569]
              shift-right: [w2563] -> w2522
              shift-left: T4 [] -> [w2564]
              i -> [w2568]
              n1288 = Index Array(array=w2569, index (col)=w2568) -> (element=w2567:dbl[])  [unwired: 1 in]
              n1289 = Bundle("TimeArray"=w2565, "DataArray"=w2567) -> (w2566:T35)  [unwired: 1 in]
              n1290 = Build Array (concatenate)(w2564, w2566) -> (w2563:T4)
            }
            "Graph DMMs 2" <- w2522
            "Graph DMMs 1" <- w2522
            "Graph DMMs 3" <- w2522
            n1291 = Index Array(array=w2520, index #1="index T_2", index #2="index T_ 1") -> (element #1=w2519:dbl, element #2=w2516:dbl)
            n1292 = Index Array(array=w2520, index #1="index V", index #2="index I") -> (element #1=w2529:dbl, element #2=w2528:dbl)
            n1293 = Subtract(x=w2519, y=w2516) -> (x-y=→"ƒ¢T=T_2 -T_1":dbl)
            n1294 = Multiply(x=w2529, y=w2528) -> (x*y=→"Q = I *V":dbl)
          }
          frame True {
            n1295 = local write "Initialize (DMMs)"(FALSE ("Initialize 2")) -> ()
            n1296 = local read "RUN Identifier"() -> (w2573:string)
            n1297 = local read "Base Path"() -> (w2578:path)
            n1298 = call-dynamic "DMMs_initialize.vi"("DMMsConfig (variables)"="DMMsConfig (variables)", "DMMsConfig"="DMMsConfig", "InstName"="InstName DMMs", "error in (no error)"=w2577, "base path"=w2578, "RunIdentifier"=w2573, "DMMsData in"=w2581) -> ("error out"=w2574:errorcluster, "DMMsLabels"=w2575:string[], "FileName"=→"DMMFileName":string, "DMMsData out"=w2580:refnum<class "DMMsData.lvclass">, "VariableSources"=→"VariableSources":T12)
            "DMMsLabels" <- w2575
            n1299 = stacked-sequence {
              tunnel: w2575 -> [w2583 w2606 w2629]
              frame #0 {
                n1300 = Array Size(array=w2583) -> (size(s)=w2592:i32)
                n1301 = control-ref of="Graph DMMs 1"() -> (w2589:refnum<vi>)
                n1302 = property class="XYGraph (strict)"(reference=w2589, error in=errorcluster {"status"=FALSE, "code"=0, "source"=""} ("error in (no error)")) -> (reference out=w2585:refnum<vi>, error out=w2588:errorcluster, "LegNumRows"=w2590:u32)
                n1303 = for {
                  N: w2590 -> [_]
                  shift-right: [w2601] -> w2591
                  shift-left: w2588 -> [w2602]
                  tunnel: w2585 -> [w2600]
                  tunnel: [w2599] -> w2584 mode=indexing
                  i -> [w2604]
                  n1304 = property class="XYGraph (strict)"(reference=w2600, error in=w2602, "Active Plot"=w2604, "Plot.Plot Name"="") -> (reference out=w2599:refnum<vi>, error out=w2601:errorcluster)
                }
                n1305 = for {
                  N: w2592 -> [_]
                  shift-right: [w2596] -> w2586
                  shift-left: w2591 -> [w2597]
                  tunnel: w2584 -> [w2594] mode=indexing
                  tunnel: w2583 -> [w2593] mode=indexing
                  i -> [w2598]
                  n1306 = property class="XYGraph (strict)"(reference=w2594, error in=w2597, "Active Plot"=w2598, "Plot.Plot Name"=w2593, "Plot.Visible?"=TRUE ("Plot.Visible")) -> (error out=w2596:errorcluster)  [unwired: 1 out]
                }
                "error out (DMM graphs)" <- w2586
              }
              frame #1 {
                n1307 = Array Size(array=w2606) -> (size(s)=w2614:i32)
                n1308 = control-ref of="Graph DMMs 2"() -> (w2609:refnum<vi>)
                n1309 = property class="XYGraph (strict)"(reference=w2609, error in=errorcluster {"status"=FALSE, "code"=0, "source"=""} ("error in (no error)")) -> (reference out=w2608:refnum<vi>, error out=w2611:errorcluster, "LegNumRows"=w2612:u32)
                n1310 = for {
                  N: w2612 -> [_]
                  shift-right: [w2623] -> w2613
                  shift-left: w2611 -> [w2624]
                  tunnel: w2608 -> [w2622]
                  tunnel: [w2621] -> w2607 mode=indexing
                  i -> [w2626]
                  n1311 = property class="XYGraph (strict)"(reference=w2622, error in=w2624, "Active Plot"=w2626, "Plot.Plot Name"="") -> (reference out=w2621:refnum<vi>, error out=w2623:errorcluster)
                }
                n1312 = for {
                  N: w2614 -> [_]
                  shift-right: [w2618] -> w2605
                  shift-left: w2613 -> [w2619]
                  tunnel: w2607 -> [w2616] mode=indexing
                  tunnel: w2606 -> [w2615] mode=indexing
                  i -> [w2620]
                  n1313 = property class="XYGraph (strict)"(reference=w2616, error in=w2619, "Active Plot"=w2620, "Plot.Plot Name"=w2615, "Plot.Visible?"=TRUE ("Plot.Visible")) -> (error out=w2618:errorcluster)  [unwired: 1 out]
                }
                n1314 = local write "error out (DMM graphs)"(w2605) -> ()
              }
              frame #2 {
                n1315 = Array Size(array=w2629) -> (size(s)=w2636:i32)
                n1316 = control-ref of="Graph DMMs 3"() -> (w2627:refnum<vi>)
                n1317 = property class="XYGraph (strict)"(reference=w2627, error in=errorcluster {"status"=FALSE, "code"=0, "source"=""} ("error in (no error)")) -> (reference out=w2631:refnum<vi>, error out=w2633:errorcluster, "LegNumRows"=w2634:u32)
                n1318 = for {
                  N: w2634 -> [_]
                  shift-right: [w2645] -> w2635
                  shift-left: w2633 -> [w2646]
                  tunnel: w2631 -> [w2644]
                  tunnel: [w2643] -> w2630 mode=indexing
                  i -> [w2648]
                  n1319 = property class="XYGraph (strict)"(reference=w2644, error in=w2646, "Active Plot"=w2648, "Plot.Plot Name"="") -> (reference out=w2643:refnum<vi>, error out=w2645:errorcluster)
                }
                n1320 = for {
                  N: w2636 -> [_]
                  shift-right: [w2640] -> w2628
                  shift-left: w2635 -> [w2641]
                  tunnel: w2630 -> [w2638] mode=indexing
                  tunnel: w2629 -> [w2637] mode=indexing
                  i -> [w2642]
                  n1321 = property class="XYGraph (strict)"(reference=w2638, error in=w2641, "Active Plot"=w2642, "Plot.Plot Name"=w2637, "Plot.Visible?"=TRUE ("Plot.Visible")) -> (error out=w2640:errorcluster)  [unwired: 1 out]
                }
                n1322 = local write "error out (DMM graphs)"(w2628) -> ()
              }
            }
          }
        }
        "error out (DMMs)" <- w2509
      }
    }
    n1323 = Get Notifier Status(notifier=w2498, error in (no error)=w2497) -> (current notification=w2495:bool, error out=w2496:errorcluster)  [unwired: 3 out]
    "cycle # (DMMs)" <- w2499
  }
  n1324 = call-dynamic "USBData_terminate.vi"("error in (no error)"=w24, "USBData in"=w25) -> ("error out"=w26:errorcluster)  [unwired: 8 in, 1 out]
  n1325 = local write "error out (USB6210)"(w26) -> ()
  n1326 = call-dynamic "DMMs_terminate.vi"("error in (no error)"=w7, "DMMsData in"=w8) -> ("error out"=→"error out (DMMs) 2":errorcluster)  [unwired: 8 in, 1 out]
  n1327 = call-dynamic "USBData_terminate.vi"("error in (no error)"=w39, "USBData in"=w40) -> ("error out"=w41:errorcluster)  [unwired: 8 in, 1 out]
  n1328 = call-dynamic "LSI336Data_terminate.vi"("error in (no error)"=w30, "LSI336Data in"=w31) -> ("error out"=w29:errorcluster)  [unwired: 8 in, 1 out]
  n1329 = Merge Errors(w11, w13) -> (w14:errorcluster)
  n1330 = local write "error out (USB6210)"(w41) -> ()
  n1331 = local write "error out (LSI336)"(w29) -> ()
  n1332 = call "LSI218Data_terminate.vi"("error in (no error)"=w34, "LSI218Data in"=w35) -> ("error out"=w33:errorcluster)  [unwired: 8 in, 1 out]
  n1333 = Release Notifier(notifier=w12, error in (no error)=w14) -> (error out=→"error out (notifier)":errorcluster)  [unwired: 1 in, 2 out]
  n1334 = local write "error out (LSI218)"(w33) -> ()
